vi "MasterAcquisitionFile_2P_Test.vi"() -> ()   [LabVIEW 2020]
uses:
  <vilib>/userDefined/High Color/IMAQdx.ctl
  <vilib>/vision/driver/IMAQdx.llb/IMAQdx Camera Control Mode.ctl
  <vilib>/vision/driver/IMAQdx.llb/IMAQdx Acquisition Mode.ctl
  <vilib>/vision/driver/IMAQdx.llb/IMAQdx Buffer Number Mode.ctl
  <vilib>/DAQmx/write.llb/DAQmx Write (Digital 1D Wfm NChan NSamp).vi
  <vilib>/DAQmx/read.llb/DAQmx Read (Analog 1D Wfm NChan NSamp).vi
  <vilib>/Waveform/DWDTOps.llb/DWDT Digital to Boolean Array.vi
  <vilib>/DAQmx/create/channels.llb/DAQmx Create Channel (DO-Digital Output).vi
  <vilib>/DAQmx/configure/timing.llb/DAQmx Timing (Sample Clock).vi
  <vilib>/Waveform/DWDTOps.llb/DWDT Boolean Array to Digital.vi
  <vilib>/Waveform/DWDTOps.llb/DWDT Uncompress Digital.vi
  <vilib>/DAQmx/miscellaneous.llb/DAQmx Fill In Error Info.vi
  <vilib>/DAQmx/create/channels.llb/DAQmx Create Channel (AI-Voltage-Basic).vi
  <vilib>/DAQmx/configure/trigger.llb/DAQmx Start Trigger (Digital Edge).vi
  <vilib>/DAQmx/create/channels.llb/DAQmx Create Channel (CO-Pulse Generation-Frequency).vi
  <vilib>/DAQmx/configure/timing.llb/DAQmx Timing (Implicit).vi
  <vilib>/DAQmx/read.llb/DAQmx Read (Digital 1D Bool 1Chan 1Samp).vi
  <vilib>/DAQmx/create/channels.llb/DAQmx Create Channel (DI-Digital Input).vi
  <vilib>/vision/driver/NI_Vision_Acquisition_Software.lvlib
  <resource>/objmgr/imaqdx.rc
  <resource>/objmgr/daqmx.rc
panel:
  in  "Analog Input Channels":tag="Dev2/ai0:3"
  out "Auditory":bool
  out "RPad":bool
  out "LPad":bool
  in  "Sol Stim Parameters":cluster{"Fs":dbl, "Samples":dbl}
  in  "LED Stim Parameters":cluster{"Fs":dbl, "Samples":dbl}
  in  "Generate Stimuli":bool=TRUE
  in  "Sol Duty Cycle (%)":dbl=50.0
  in  "Sol Freq":dbl=5.0
  in  "Sol Dur (s)":dbl=5.0
  in  "LED Duty Cycle (%)":dbl=10.0
  in  "LED Freq":dbl=10.0
  in  "LED Dur (s)":dbl=2.0
  out "Stimulus Order":digitalwaveform[](graph)=[{"t0"=timestamp(0 s since 1904-01-01), "dt"=5e-05, "Y"={"transitions"=[], "data"=array19221000x1[19221000 elements]}}, {"t0"=timestamp(0 s since 1904-01-01), "dt"=5e-05, "Y"={"transitions"=[], "data"=array19221000x1[19221000 elements]}}, {"t0"=timestamp(0 s since 1904-01-01), "dt"=5e-05, "Y"={"transitions"=[], "data"=array19221000x1[19221000 elements]}}]
  out "Solenoid Stim":digitalwaveform(graph)={"t0"=timestamp(0 s since 1904-01-01), "dt"=5e-05, "Y"={"transitions"=[], "data"=array100000x1[100000 elements]}}
  in  "Trial Offset (s)":dbl=45.0
  in  "Interstim (s)":dbl=45.0
  in  "Right Pad":dbl=1.0
  in  "Left Pad":dbl=1.0
  in  "Auditory":dbl=1.0
  in  "LED":dbl
  out "?":T1(plugin-control)
  out "MSCan Cam Fs":dbl(knob) scale=0.0..200.0
  out "MScan Cam":bool
  out "?":T1(plugin-control)
  in  "stop":bool
  out "?":T1(plugin-control)
  out "Behavior Cam Fs":dbl(knob) scale=0.0..200.0
  out "Behav Cam":bool
  out "Complete":bool
  out "Whisk Cam":bool
  out "Analog":bool
  out "MScan Trig":bool
  out "?":bool[](array[boolean])=[TRUE]
  out "Hexadecimal Data":u32=1 format="%x"
  out "Time Elapsed (Min)":cluster{dbl, dbl}(slide)={16.0, 0.0} scale=0.0..16.0 scale format="%#_2g"
  out "Whisker Camera":bool
  out "Analog Data":bool
  out "Analog Samples":i32=15417328
  in  "Device Analog Channel Labels":string[](array[string])=["forceSensor", "LPadSol", "RPadSol", "AudSol", "", "", "", ""]
  in  "?":cluster{"Analog Fs":u16}={"Analog Fs"=20000} {"Analog Fs" format="%0.0f"}
  in  "?":cluster{"WhiskerCam Fs":u16}={"WhiskerCam Fs"=150}
  out "Notes Size":i32=7
  out "Notes Reversed":string[](array[string])=["Experimenter", "Animal ID", "Isoflurane time", "Amplifier Gain", "Session ID", "Hemisphere", "Solenoid PSI"]
  out "Notes Array":string[](array[string])=["Solenoid PSI", "Hemisphere", "Session ID", "Amplifier Gain", "Isoflurane time", "Animal ID", "Experimenter"]
  in  "Notes:":T2={"Experimenter"="Kevin\n", "Animal ID"="T192", "Isoflurane time"="1145", "Amplifier Gain"="10000", "Session ID"="Imaging Session One", "Hemisphere"="RH", "Solenoid PSI"="10"}
  in  "Target Path":path=path "C:/Users/klt8/Documents" caption="Final Saved File Location"
  out "Dropped":u32(slide) caption="WhiskerCam" scale=0.0..150.0
  out "Current File Name":string="210517_13_39_46"
  in  "Time (min)":dbl(knob)=16.0 min=0.5 max=20.0 step=0.5 scale=0.0..20.0 scale format="%#_3g"
  in  "Temp Path":path=path "C:/Users/klt8/Documents/LabVIEW Temp Files" caption="Temporary File Path"
  out "Last Whisk Buffer":u32=115624
  out "Whisker Cam Fs":dbl(knob) scale=0.0..200.0 scale format="%#1_6g"
  # "Notes"
  # "Dropped Frames"
  # "LPAD"
  # "RPAD"
  # "AUD"
  # "Analog\nFs"
  # "Whisker\nFs"
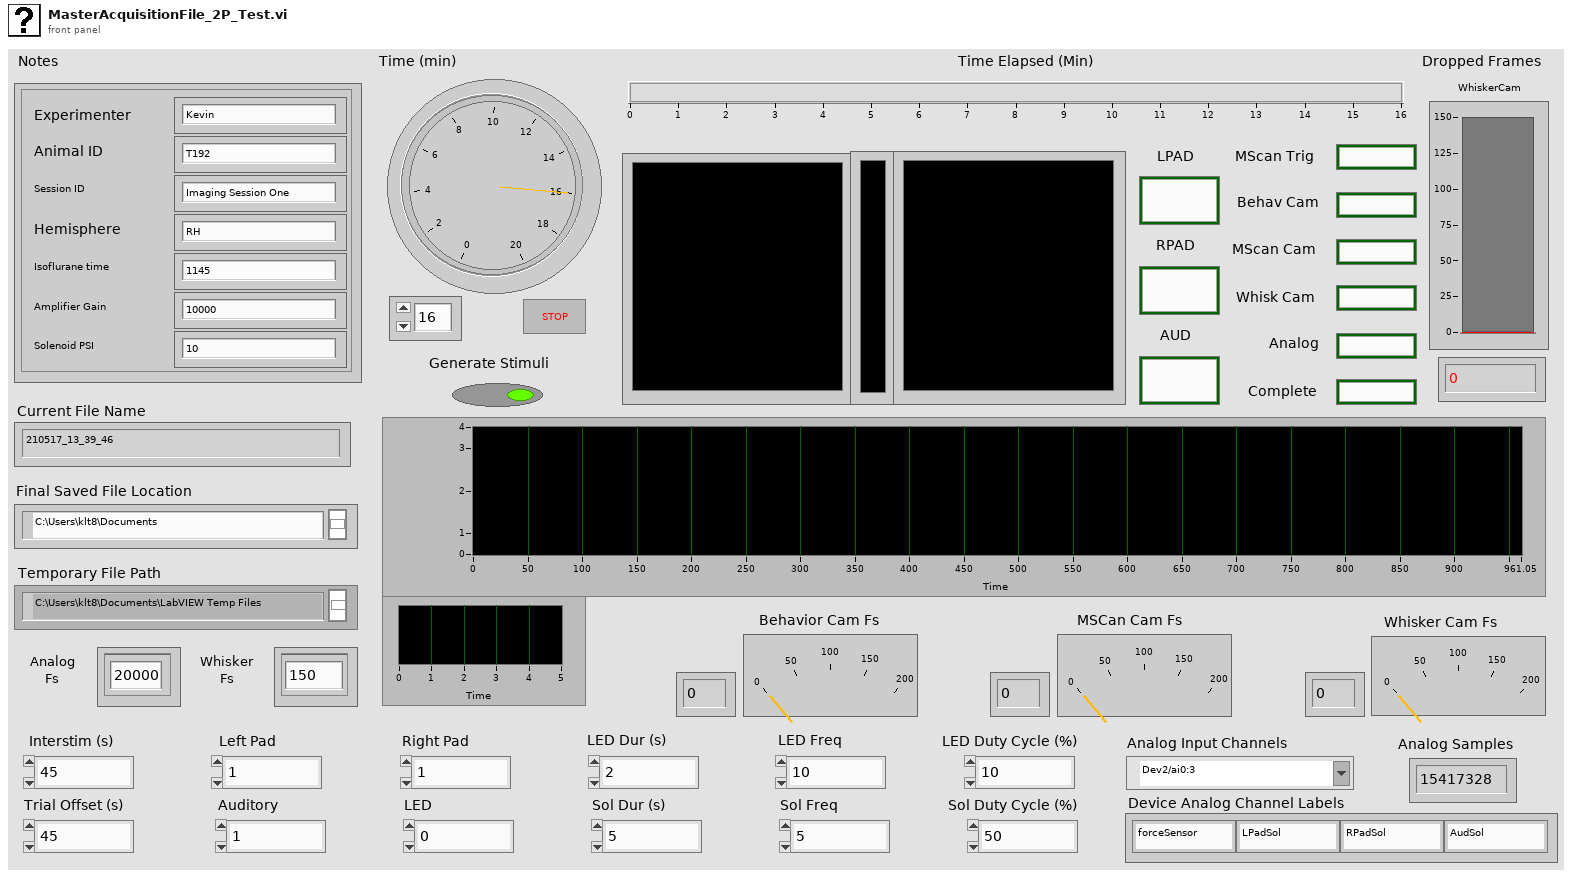
[diagram p1: front panel]
types:
  T1 = typedef "IMAQ Image.ctl" = refnum<image>
  T2 = cluster{"Experimenter":string, "Animal ID":string, "Isoflurane time":string, "Amplifier Gain":string, "Session ID":string, "Hemisphere":string, "Solenoid PSI":string}
  T3 = typedef "IMAQdx.ctl" = refnum<k21>
  T4 = typedef "NI_Vision_Acquisition_Software.lvlib/IMAQdx Camera Control Mode.ctl" = enum32{"Controller", "Listener"}
  T5 = enum16{"open", "open or create", "create or replace", "create", "open (read-only)"}
  T6 = enum16{"open", "replace", "create", "open or create", "replace or create", "replace or create with confirmation"}
  T7 = typedef "NI_Vision_Acquisition_Software.lvlib/IMAQdx Acquisition Mode.ctl" = enum32{"One Shot", "Continuous"}
  T8 = enum16{"big-endian, network order", "native, host order", "little-endian"}
  T9 = typedef "NI_Vision_Acquisition_Software.lvlib/IMAQdx Buffer Number Mode.ctl" = enum32{"Next", "Last", "Buffer Number", "Every", "Last New"}
  T10 = typedef "Image Type" = u32
  T11 = typedef "IMAQ AVI2 Refnum.ctl" = refnum<k20>
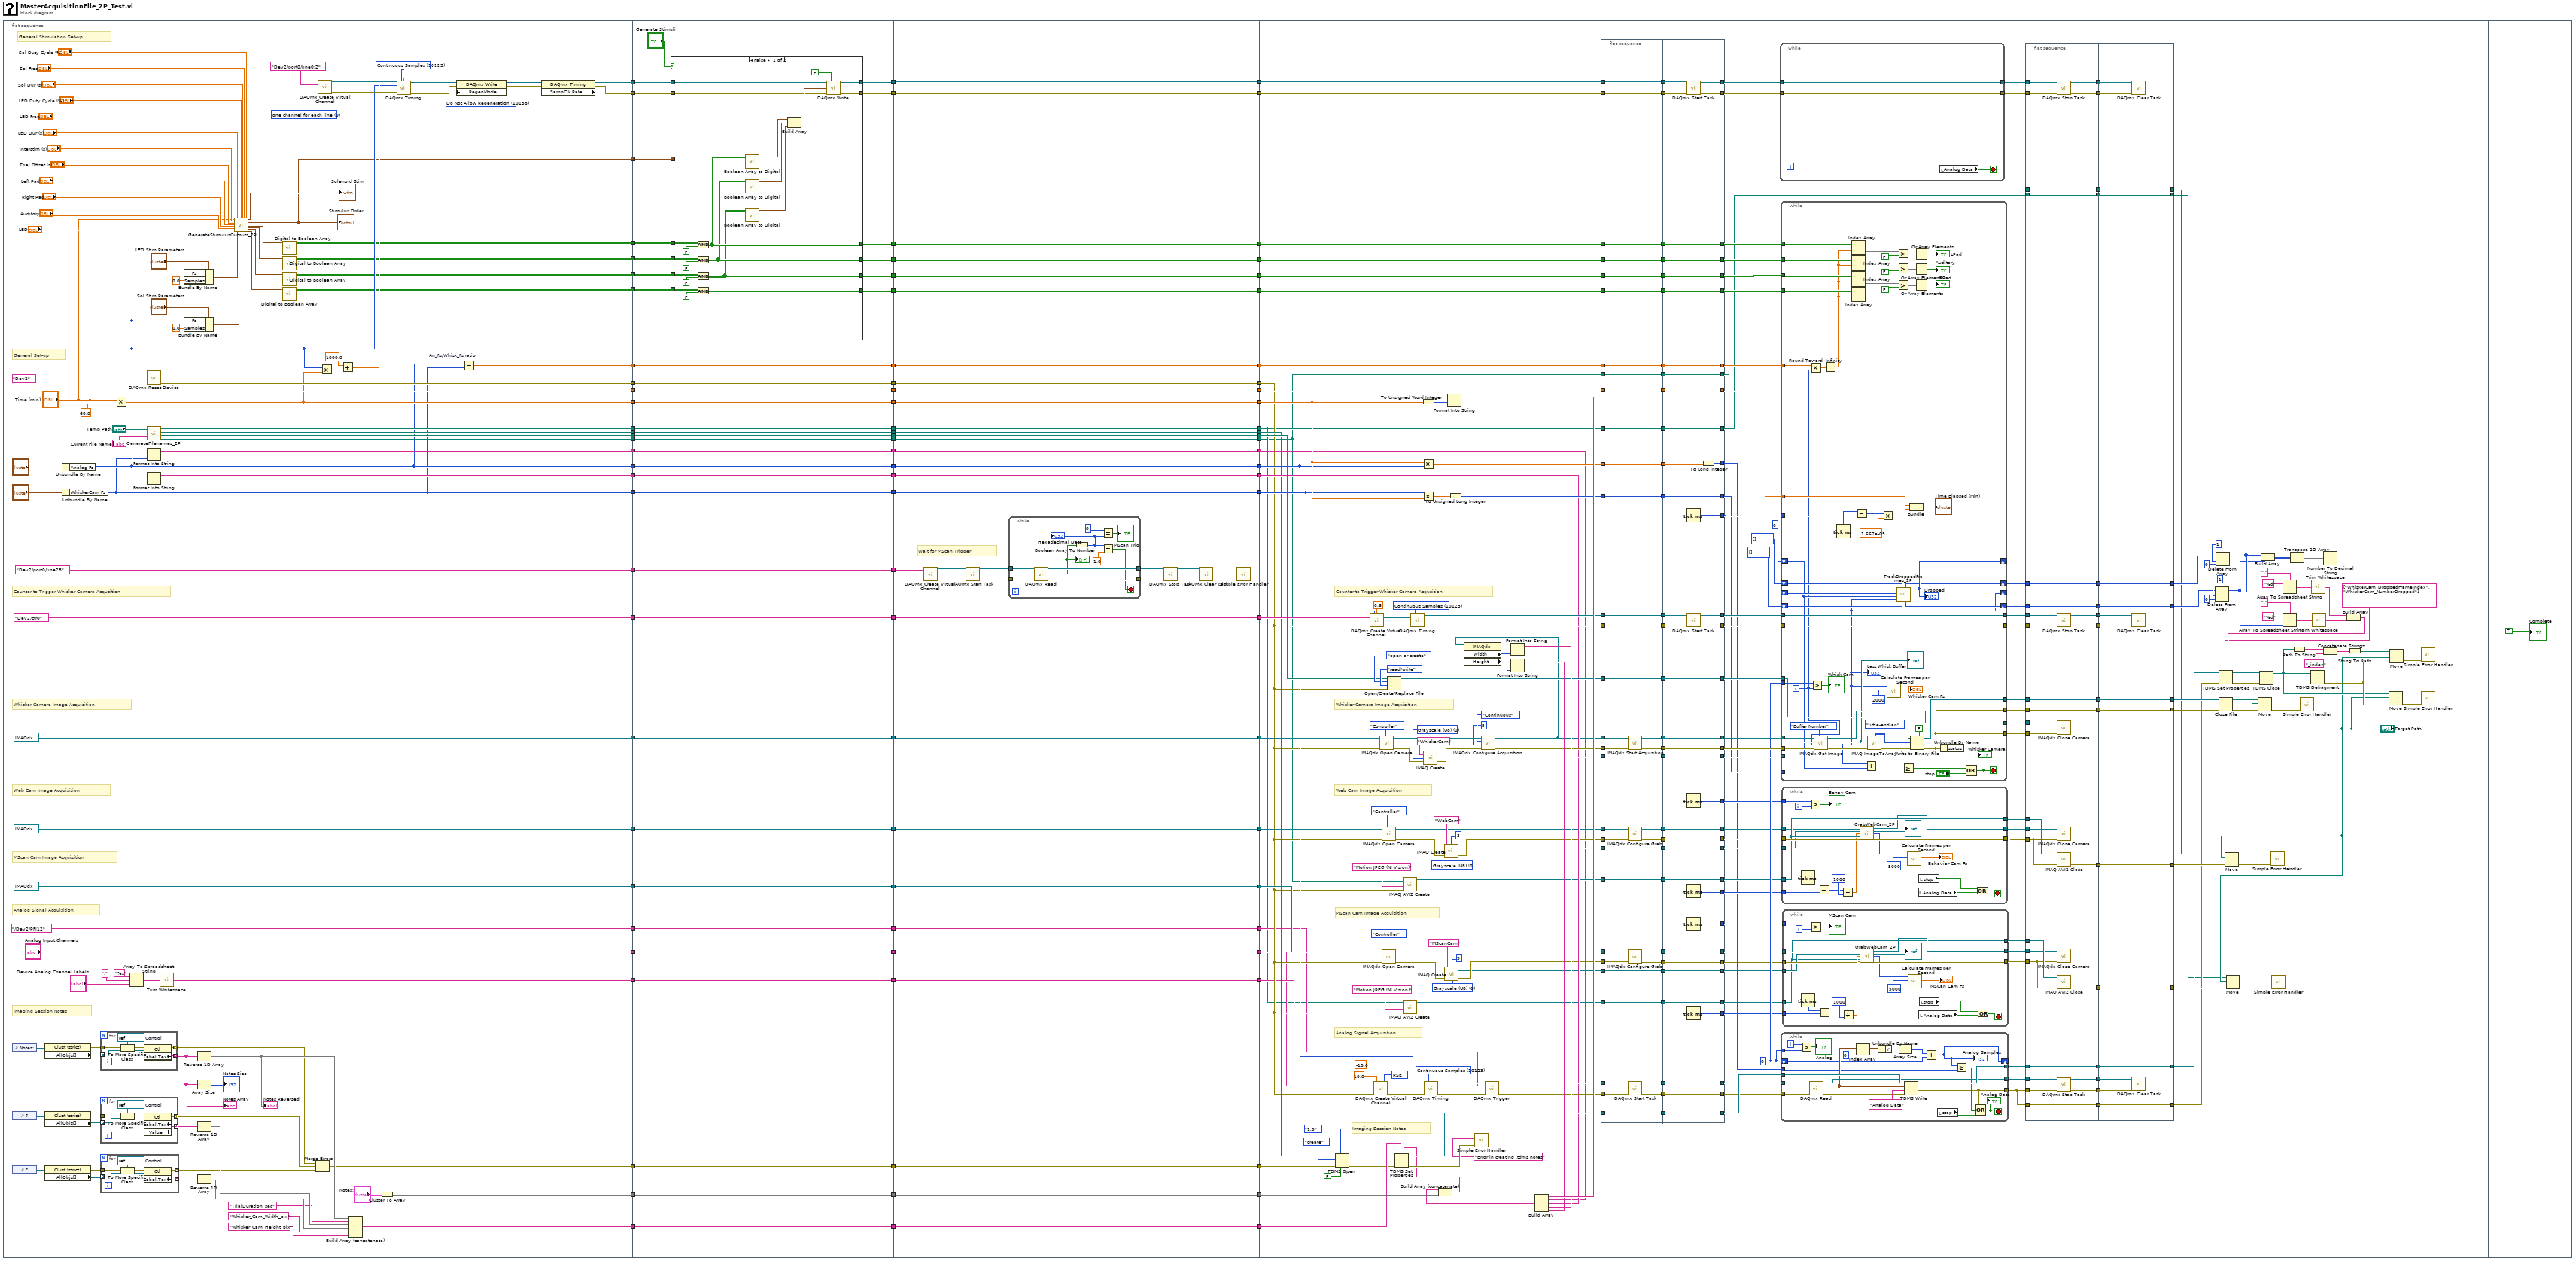
[diagram p0: block diagram]
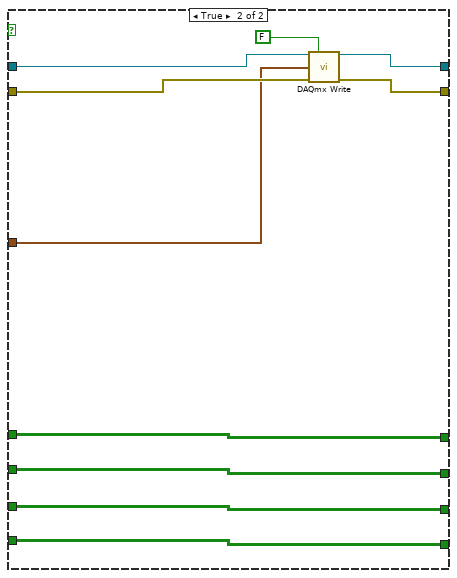
[diagram p2: hidden frame]
diagram:
  n1 = flat-sequence {
    tunnel: [tag "/Dev2/PFI12" ("Whisk Cam Trigger")] -> w62
    tunnel: [w109] -> w60
    tunnel: ["Time (min)"] -> w58
    tunnel: [w156] -> w56
    tunnel: [w155] -> w54
    tunnel: [w107] -> w52
    tunnel: [w106] -> w50
    tunnel: [w154] -> w48
    tunnel: [tag "Dev2/ctr0" ("Whisk Cam Counter")] -> w46
    tunnel: [w153] -> w44
    tunnel: ["Analog Input Channels"] -> w42
    tunnel: [T3 "cam1" ("Whisker Cam ID")] -> w40
    tunnel: [w152] -> w38
    tunnel: [w150] -> w36
    tunnel: [w151] -> w34
    tunnel: [T3 "cam2" ("WebCam ID")] -> w32
    tunnel: [tag "Dev2/port0/line28" ("MScan Trigger")] -> w30
    tunnel: [w147] -> w28
    tunnel: [w146] -> w26
    tunnel: [w145] -> w24
    tunnel: [T3 "cam7" ("WebCam ID 2")] -> w22
    tunnel: [w144] -> w20
    tunnel: [w105] -> w12
    tunnel: [w94] -> w10
    tunnel: [w93] -> w9
    tunnel: [w92] -> w8
    tunnel: [w91] -> w7
    tunnel: [w90] -> w6
    tunnel: [w89] -> w5
    tunnel: [w88] -> w4
    tunnel: w62 -> [w244]
    tunnel: [w244] -> w61
    tunnel: w60 -> [w243]
    tunnel: [w243] -> w59
    tunnel: w58 -> [w242]
    tunnel: [w242] -> w57
    tunnel: w56 -> [w241]
    tunnel: [w241] -> w55
    tunnel: w54 -> [w240]
    tunnel: [w240] -> w53
    tunnel: w52 -> [w239]
    tunnel: [w239] -> w51
    tunnel: w50 -> [w238]
    tunnel: [w238] -> w49
    tunnel: w48 -> [w237]
    tunnel: [w237] -> w47
    tunnel: w46 -> [w236]
    tunnel: [w236] -> w45
    tunnel: w44 -> [w235]
    tunnel: [w235] -> w43
    tunnel: w42 -> [w234]
    tunnel: [w234] -> w41
    tunnel: w40 -> [w233]
    tunnel: [w233] -> w39
    tunnel: w38 -> [w232]
    tunnel: [w232] -> w37
    tunnel: w36 -> [w231]
    tunnel: [w231] -> w35
    tunnel: w34 -> [w230]
    tunnel: [w230] -> w33
    tunnel: w32 -> [w229]
    tunnel: [w229] -> w31
    tunnel: w30 -> [w228]
    tunnel: [w228] -> w29
    tunnel: w28 -> [w227]
    tunnel: [w227] -> w27
    tunnel: w26 -> [w226]
    tunnel: [w226] -> w25
    tunnel: w24 -> [w225]
    tunnel: [w225] -> w23
    tunnel: w22 -> [w224]
    tunnel: [w224] -> w21
    tunnel: w20 -> [w223]
    tunnel: [w223] -> w19
    tunnel: [w214] -> w18
    tunnel: [w213] -> w17
    tunnel: [w212] -> w16
    tunnel: [w211] -> w15
    tunnel: [w210] -> w14
    tunnel: [w209] -> w13
    tunnel: w12 -> [w222]
    tunnel: [w222] -> w11
    tunnel: w10 -> [w221]
    tunnel: w9 -> [w220]
    tunnel: w8 -> [w219]
    tunnel: w7 -> [w218]
    tunnel: w6 -> [w217]
    tunnel: w5 -> [w216]
    tunnel: w4 -> [w215]
    tunnel: [w293] -> w87
    tunnel: [w304] -> w86
    tunnel: [w305] -> w85
    tunnel: [w306] -> w84
    tunnel: [w307] -> w83
    tunnel: [w294] -> w82
    tunnel: [w308] -> w81
    tunnel: [w309] -> w80
    tunnel: [w310] -> w79
    tunnel: [w311] -> w78
    tunnel: [w312] -> w77
    tunnel: [w313] -> w76
    tunnel: w61 -> [w278]
    tunnel: w59 -> [w313]
    tunnel: w57 -> [w312]
    tunnel: w55 -> [w311]
    tunnel: w53 -> [w310]
    tunnel: w51 -> [w309]
    tunnel: w49 -> [w308]
    tunnel: w47 -> [w294]
    tunnel: w45 -> [w307]
    tunnel: w43 -> [w276]
    tunnel: w41 -> [w277]
    tunnel: w39 -> [w306]
    tunnel: w37 -> [w305]
    tunnel: w35 -> [w304]
    tunnel: w33 -> [w293]
    tunnel: [w291] -> w75
    tunnel: w31 -> [w291]
    tunnel: w29 -> [w292]
    tunnel: w27 -> [w290]
    tunnel: [w290] -> w74
    tunnel: w25 -> [w289]
    tunnel: w23 -> [w288]
    tunnel: [w289] -> w73
    tunnel: [w288] -> w72
    tunnel: w21 -> [w287]
    tunnel: [w287] -> w71
    tunnel: w19 -> [w286]
    tunnel: [w286] -> w70
    tunnel: [w285] -> w69
    tunnel: w18 -> [w285]
    tunnel: [w284] -> w68
    tunnel: w17 -> [w284]
    tunnel: [w283] -> w67
    tunnel: w16 -> [w283]
    tunnel: [w282] -> w66
    tunnel: w15 -> [w282]
    tunnel: [w281] -> w65
    tunnel: w14 -> [w281]
    tunnel: w13 -> [w280]
    tunnel: [w280] -> w64
    tunnel: [w279] -> w63
    tunnel: w11 -> [w279]
    tunnel: [w278] -> w3
    tunnel: [w277] -> w2
    tunnel: [w276] -> w1
    tunnel: w87 -> [w468]
    tunnel: w86 -> [w474]
    tunnel: w85 -> [w416]
    tunnel: w84 -> [w473]
    tunnel: w83 -> [w472]
    tunnel: w82 -> [w471]
    tunnel: w81 -> [w441]
    tunnel: w80 -> [w431]
    tunnel: w79 -> [w470]
    tunnel: w78 -> [w430]
    tunnel: w77 -> [w465]
    tunnel: w76 -> [w469]
    tunnel: w75 -> [w456]
    tunnel: w74 -> [w348]
    tunnel: w73 -> [w437]
    tunnel: w72 -> [w435]
    tunnel: w71 -> [w418]
    tunnel: w70 -> [w350]
    tunnel: w69 -> [w370]
    tunnel: w68 -> [w368]
    tunnel: w67 -> [w374]
    tunnel: w66 -> [w373]
    tunnel: w65 -> [w372]
    tunnel: w64 -> [w371]
    tunnel: w63 -> [w389]
    tunnel: w3 -> [w354]
    tunnel: w2 -> [w352]
    tunnel: w1 -> [w353]
    frame #0 {
      w124 = 10158 items=["Allow Regeneration"=10097, "Do Not Allow Regeneration"=10158] ("RegenMode")
      w125 = 10123 items=["Finite Samples"=10178, "Continuous Samples"=10123, "Hardware Timed Single Point"=12522] ("sample mode")
      w128 = 0 items=["one channel for each line", "one channel for all lines"] ("line grouping")
      # "General Stimulation Set-up"
      # "MScan Cam Image Acquisition"
      # "General Set-up"
      # "Whisker Camera Image Acquisition"
      # "Imaging Session Notes"
      # "Counter to Trigger Whisker Camera Acqusition"
      # "Web Cam Image Acquisition"
      # "Analog Signal Acquisition"
      n2 = control-ref of="Notes:"() -> (w172:refnum<vi>)
      n3 = control-ref of="?"() -> (w170:refnum<vi>)
      n4 = control-ref of="?"() -> (w163:refnum<vi>)
      n5 = property class="Clust (strict)"(reference=w172) -> (error out=w171:errorcluster, "AllObjs[]"=w173:refnum<vi>[])  [unwired: 1 in, 1 out]
      n6 = property class="Clust (strict)"(reference=w170) -> (error out=w168:errorcluster, "AllObjs[]"=w169:refnum<vi>[])  [unwired: 1 in, 1 out]
      n7 = property class="Clust (strict)"(reference=w163) -> (error out=w164:errorcluster, "AllObjs[]"=w166:refnum<vi>[])  [unwired: 1 in, 1 out]
      n8 = Unbundle By Name("?") -> ("Analog Fs"=w107:u16)
      n9 = Unbundle By Name("?") -> ("WhiskerCam Fs"=w106:u16)
      n10 = for {
        tunnel: [w191] -> w178 mode=indexing
        tunnel: w173 -> [w190] mode=indexing
        tunnel: w171 -> [w189]
        tunnel: [w187] -> w177 mode=indexing
        w192 = refnum<vi> refnum  # Control
        n11 = To More Specific Class(target class=w192, reference=w190, error in=w189) -> (specific class reference=w193:refnum<vi>, error out=w188:errorcluster)
        n12 = property class="Ctl"(reference=w193, error in=w188) -> (error out=w187:errorcluster, "Label.Text"=w191:string)  [unwired: 1 out]
      }
      "Notes Array" <- w178
      n13 = for {
        tunnel: [w198] -> w167 mode=indexing
        tunnel: w169 -> [w197] mode=indexing
        tunnel: w168 -> [w196]
        tunnel: [w194] -> w176 mode=indexing
        w199 = refnum<vi> refnum  # Control
        n14 = To More Specific Class(target class=w199, reference=w197, error in=w196) -> (specific class reference=w200:refnum<vi>, error out=w195:errorcluster)
        n15 = property class="Ctl" props=["Label", "Text", "Value"](reference=w200, error in=w195) -> (error out=w194:errorcluster, "Label.Text"=w198:string)  [unwired: 2 out]
      }
      n16 = for {
        tunnel: [w205] -> w165 mode=indexing
        tunnel: w166 -> [w204] mode=indexing
        tunnel: w164 -> [w203]
        tunnel: [w201] -> w175 mode=indexing
        w206 = refnum<vi> refnum  # Control
        n17 = To More Specific Class(target class=w206, reference=w204, error in=w203) -> (specific class reference=w207:refnum<vi>, error out=w202:errorcluster)
        n18 = property class="Ctl"(reference=w207, error in=w202) -> (error out=w201:errorcluster, "Label.Text"=w205:string)  [unwired: 1 out]
      }
      n19 = Multiply(x="Time (min)", y=60.0) -> (x*y=w109:dbl)
      n20 = Array To Spreadsheet String(delimiter (Tab)=",", array="Device Analog Channel Labels", 3:"%s" ("format string")) -> (spreadsheet string=w180:string)
      n21 = call <vilib>:"DAQmx Reset Device.vi"("device in"=tag "Dev2" ("NI Board")) -> ("error out"=w152:errorcluster)  [unwired: 14 in]
      n22 = call "GenerateFilenames_2P.vi"("path"="Temp Path") -> ("WebCam Path"=w147:path, "Basler Path"=w150:path, "TDMS Path"=w145:path, "MScan Path"=w144:path, "Analog file name"=→"Current File Name":string)  [unwired: 2 in]
      n23 = Format Into String(w106) -> (resulting string=w156:string)  [unwired: 3 in, 1 out]
      n24 = Format Into String(w107) -> (resulting string=w155:string)  [unwired: 3 in, 1 out]
      n25 = call <vilib>:"Trim Whitespace.vi"("string"=w180) -> ("trimmed string"=w153:string)  [unwired: 1 in]
      n26 = Bundle By Name(cluster="LED Stim Parameters", "Fs"=w107, "Samples"=0.0) -> (w114:cluster{"Fs":dbl, "Samples":dbl})
      n27 = Bundle By Name(cluster="Sol Stim Parameters", "Fs"=w107, "Samples"=0.0) -> (w113:cluster{"Fs":dbl, "Samples":dbl})
      n28 = Reverse 1D Array(array=w178) -> (reversed array=w179:string[])
      "Notes Reversed" <- w179
      n29 = Array Size(array=w178) -> (size(s)=→"Notes Size":i32)
      n30 = Reverse 1D Array(array=w167) -> (reversed array=w185:string[])
      n31 = Reverse 1D Array(array=w165) -> (reversed array=w186:string[])
      n32 = call "GenerateStimulusOutputs_2P.vi"("Trial duration (min)"="Time (min)", "Rest duration(s)"="Interstim (s)", "trial offset (s)"="Trial Offset (s)", "Left Pad"="Left Pad", "Right Pad"="Right Pad", "Auditory"="Auditory", "LED"="LED", "LED Stim Duration (s)"="LED Dur (s)", "LED Stim Parameters"=w114, "LED Frequency"="LED Freq", "Sol Stim Parameters"=w113, "LED duty cycle (%)"="LED Duty Cycle (%)", "Sol Stim Duration (s)"="Sol Dur (s)", "Sol Frequency"="Sol Freq", "Sol Duty Cycle (%)"="Sol Duty Cycle (%)") -> ("Solenoid Stim Waveforms"=→"Solenoid Stim":digitalwaveform, "Stimulus Digital Outputs"=w90:digitalwaveform[], "Left Pad Out"=w103:digitalwaveform, "Auditory Out"=w130:digitalwaveform, "Right Pad Out"=w129:digitalwaveform, "LED Out"=w108:digitalwaveform)  [unwired: 7 in]
      "Stimulus Order" <- w90
      n33 = call-poly <vilib>:"Digital to Boolean Array.vi"("digital waveform"=w103) -> ("boolean array"=w89:bool[][])  [unwired: 9 in, 1 out]
      n34 = call-poly <vilib>:"Digital to Boolean Array.vi"("digital waveform"=w130) -> ("boolean array"=w92:bool[][])  [unwired: 9 in, 1 out]
      n35 = call-poly <vilib>:"Digital to Boolean Array.vi"("digital waveform"=w129) -> ("boolean array"=w91:bool[][])  [unwired: 9 in, 1 out]
      n36 = call-poly <vilib>:"Digital to Boolean Array.vi"("digital waveform"=w108) -> ("boolean array"=w88:bool[][])  [unwired: 9 in, 1 out]
      n37 = Merge Errors(w177, w176, w175) -> (w146:errorcluster)
      n38 = call-poly <vilib>:"DAQmx Create Virtual Channel.vi"("lines"=tag "Dev2/port0/line0:2", "line grouping"=w128) -> ("task out"=w127:refnum<k21>, "error out"=w126:errorcluster)  [unwired: 12 in]
      n39 = Multiply(x=w107, y=w109) -> (x*y=w112:dbl)
      n40 = Add(x=1000.0, y=w112) -> (x+y=w110:dbl)
      n41 = Build Array (concatenate)(w179, "TrialDuration_sec", w185, w186, "Whisker_Cam_Width_pix", "Whisker_Cam_Height_pix") -> (w151:string[])
      n42 = Cluster To Array(cluster="Notes:") -> (array=w154:string[])
      n43 = call-poly <vilib>:"DAQmx Timing.vi"("task/channels in"=w127, "sample mode"=w125, "samples per channel"=w110, "rate"=w107, "error in"=w126) -> ("task out"=w121:refnum<k21>, "error out"=w120:errorcluster)  [unwired: 9 in]
      n44 = property class="DAQmx Write"(reference=w121, error in=w120, "RegenMode"=w124) -> (reference out=w122:refnum<k21>, error out=w123:errorcluster)
      n45 = Divide "An_Fs/Whisk_Fs ratio"(x=w107, y=w106) -> (x/y=w105:dbl)
      n46 = property class="DAQmx Timing" props=["SampClk.Rate"](reference=w122, error in=w123) -> (reference out=w94:refnum<k21>, error out=w93:errorcluster)  [unwired: 1 out]
    }
    frame #1 {
      n47 = case shown="False" "Generate Stimuli" {
        tunnel: w221 -> [w252 w275]
        tunnel: w220 -> [w251 w274]
        tunnel: [w249 w273] -> w214
        tunnel: [w250 w272] -> w213
        tunnel: w219 -> [w264 w271]
        tunnel: w218 -> [w265 w270]
        tunnel: [w248 w268] -> w212
        tunnel: [w247 w271] -> w211
        tunnel: [w246 w270] -> w210
        tunnel: [w258 w267] -> w209
        tunnel: w217 -> [_ w269]
        tunnel: w216 -> [w259 w268]
        tunnel: w215 -> [w257 w267]
        frame False {
          n48 = Compound Arithmetic op=AND(w259, FALSE) -> (w248:bool[][])
          n49 = Compound Arithmetic op=AND(w264, FALSE) -> (w247:bool[][])
          n50 = Compound Arithmetic op=AND(w265, FALSE) -> (w246:bool[][])
          n51 = Compound Arithmetic op=AND(w257, FALSE) -> (w258:bool[][])
          n52 = call-poly <vilib>:"Boolean Array to Digital.vi"("boolean array"=w248) -> ("digital waveform"=w255:digitalwaveform)  [unwired: 9 in, 1 out]
          n53 = call-poly <vilib>:"Boolean Array to Digital.vi"("boolean array"=w247) -> ("digital waveform"=w254:digitalwaveform)  [unwired: 9 in, 1 out]
          n54 = call-poly <vilib>:"Boolean Array to Digital.vi"("boolean array"=w246) -> ("digital waveform"=w245:digitalwaveform)  [unwired: 9 in, 1 out]
          n55 = Build Array(w255, w254, w245) -> (w253:digitalwaveform[])
          n56 = call-poly <vilib>:"DAQmx Write.vi"("task/channels in"=w252, "auto start"=FALSE, "data"=w253, "error in"=w251) -> ("task out"=w249:refnum<k21>, "error out"=w250:errorcluster)  [unwired: 9 in, 1 out]
        }
        frame True {
          n57 = call-poly <vilib>:"DAQmx Write.vi"("task/channels in"=w275, "auto start"=FALSE, "data"=w269, "error in"=w274) -> ("task out"=w273:refnum<k21>, "error out"=w272:errorcluster)  [unwired: 9 in, 1 out]
        }
      }
    }
    frame #2 {
      # "Wait for MScan Trigger"
      n58 = call-poly <vilib>:"DAQmx Create Virtual Channel.vi"("lines"=w292) -> ("task out"=w299:refnum<k21>, "error out"=w300:errorcluster)  [unwired: 13 in]
      n59 = call <vilib>:"DAQmx Start Task.vi"("task/channels in"=w299, "error in"=w300) -> ("task out"=w303:refnum<k21>, "error out"=w302:errorcluster)  [unwired: 12 in]
      n60 = while {
        tunnel: w303 -> [w323]
        tunnel: w302 -> [w322]
        tunnel: [w320] -> w297
        tunnel: [w321] -> w298
        stop <- w315 stop-if-true
        n61 = call-poly <vilib>:"DAQmx Read.vi"("task/channels in"=w323, "error in"=w322) -> ("task out"=w321:refnum<k21>, "data"=w319:bool[], "error out"=w320:errorcluster)  [unwired: 11 in]
        "?" <- w319
        n62 = Boolean Array To Number(Boolean array=w319) -> (number=w314:u32)
        "Hexadecimal Data" <- w314
        n63 = Equal?(x=w314, y=u32 0) -> (x = y?=→"MScan Trig":bool)
        n64 = Equal?(x=w314, y=1.0) -> (x = y?=w315:bool)
      }
      n65 = call <vilib>:"DAQmx Stop Task.vi"("task/channels in"=w298, "error in"=w297) -> ("task out"=w296:refnum<k21>, "error out"=w295:errorcluster)  [unwired: 12 in]
      n66 = call <vilib>:"DAQmx Clear Task.vi"("task in"=w296, "error in"=w295) -> ("error out"=w301:errorcluster)  [unwired: 13 in]
      n67 = call <vilib>:"Simple Error Handler.vi"("error in (no error)"=w301) -> ()  [unwired: 4 in, 5 out]
    }
    frame #3 {
      w421 = T10 0 items=["Grayscale (U8)", "Grayscale (I16)", "Grayscale (SGL)", "Complex (CSG)", "RGB (U32)", "HSL (U32)", "RGB (U64)", "Grayscale (U16)"] ("Image Type")
      w460 = T10 0 items=["Grayscale (U8)", "Grayscale (I16)", "Grayscale (SGL)", "Complex (CSG)", "RGB (U32)", "HSL (U32)", "RGB (U64)", "Grayscale (U16)"] ("Image Type")
      w448 = u32 0 ("y")
      w483 = 10123 items=["Finite Samples"=10178, "Continuous Samples"=10123, "Hardware Timed Single Point"=12522] ("sample mode")
      w482 = 10083 items=["default"=-1, "RSE"=10083, "NRSE"=10078, "Differential"=10106, "Pseudodifferential"=12529] ("input terminal configuration")
      w484 = 10123 items=["Finite Samples"=10178, "Continuous Samples"=10123, "Hardware Timed Single Point"=12522] ("sample mode")
      w480 = T10 0 items=["Grayscale (U8)", "Grayscale (I16)", "Grayscale (SGL)", "Complex (CSG)", "RGB (U32)", "HSL (U32)", "RGB (U64)", "Grayscale (U16)"] ("Image Type")
      # "MScan Cam Image Acquisition"
      # "Whisker Camera Image Acquisition"
      # "Imaging Session Notes"
      # "Counter to Trigger Whisker Camera Acqusition"
      # "Web Cam Image Acquisition"
      # "Analog Signal Acquisition"
      n68 = TDMS Open(6:FALSE ("disable buffering? (T)"), 7:enum16{"1.0", "2.0"}."1.0" ("file format version (2.0)"), 8:w437, 10:T5."create" ("operation (0:open)"), 11:w435) -> (0:w434:errorcluster, 3:w433:refnum<k34>)  [unwired: 2 in]
      n69 = call-poly <vilib>:"DAQmx Create Virtual Channel.vi"("frequency"=w441, "duty cycle"=0.6, "counter"=w472, "error in"=w416) -> ("task out"=w507:refnum<k21>, "error out"=w508:errorcluster)  [unwired: 10 in]
      n70 = call-poly <vilib>:"DAQmx Create Virtual Channel.vi"("maximum value"=10.0, "minimum value"=-10.0, "input terminal configuration"=w482, "physical channels"=w352, "name to assign"=w353, "error in"=w416) -> ("task out"=w515:refnum<k21>, "error out"=w516:errorcluster)  [unwired: 8 in]
      n71 = call <vilib>:"IMAQdx Open Camera.vi"("Camera Control Mode"=IMAQdx_Camera_Control_Mode."Controller", "error in"=w416, "Session In"=w473) -> ("error out"=w505:errorcluster, "Session Out"=w504:T3)  [unwired: 7 in]
      n72 = call <vilib>:"IMAQdx Open Camera.vi"("Camera Control Mode"=IMAQdx_Camera_Control_Mode."Controller", "error in"=w416, "Session In"=w456) -> ("error out"=w457:errorcluster, "Session Out"=w455:T3)  [unwired: 7 in]
      n73 = call <vilib>:"IMAQdx Open Camera.vi"("Camera Control Mode"=IMAQdx_Camera_Control_Mode."Controller", "error in"=w416, "Session In"=w418) -> ("error out"=w419:errorcluster, "Session Out"=w413:T3)  [unwired: 7 in]
      n74 = Open/Create/Replace File(file path (use dialog)=w474, error in=w416, operation (0:open)=T6."open or create", access (0:read/write)=enum16{"read/write", "read-only", "write-only"}."read/write") -> (refnum out=w514:refnum<file>)  [unwired: 2 in, 2 out]
      n75 = call "IMAQ AVI2 Create"("error in (no error)"=w416, "Codec"="Motion JPEG (NI Vision)", "AVI Path"=w348) -> ("AVI Refnum"=w443:T11)  [unwired: 7 in, 1 out]
      n76 = call "IMAQ AVI2 Create"("error in (no error)"=w416, "Codec"="Motion JPEG (NI Vision)", "AVI Path"=w350) -> ("AVI Refnum"=w409:T11)  [unwired: 7 in, 1 out]
      n77 = call-poly <vilib>:"DAQmx Timing.vi"("task/channels in"=w507, "sample mode"=w484, "error in"=w508) -> ("task out"=w524:refnum<k21>, "error out"=w525:errorcluster)  [unwired: 11 in]
      n78 = Multiply(x=w469, y=w431) -> (x*y=w547:dbl)
      n79 = Multiply(x=w441, y=w469) -> (x*y=w548:dbl)
      n80 = To Unsigned Word Integer(number=w469) -> (unsigned 16bit integer=w537:u16)
      n81 = call "IMAQ Create"("Image Name"="WhiskerCam", "Image Type"=w480, "error in (no error)"=w505) -> ("New Image"=w540:T1, "error out"=w506:errorcluster)  [unwired: 2 in]
      n82 = call-poly <vilib>:"DAQmx Timing.vi"("task/channels in"=w515, "sample mode"=w483, "rate"=w431, "error in"=w516) -> ("task out"=w517:refnum<k21>, "error out"=w518:errorcluster)  [unwired: 10 in]
      n83 = call "IMAQ Create"("Border Size"=3, "Image Name"="WebCam", "Image Type"=w460, "error in (no error)"=w457) -> ("New Image"=w453:T1, "error out"=w454:errorcluster)  [unwired: 1 in]
      n84 = call "IMAQ Create"("Border Size"=3, "Image Name"="MScanCam", "Image Type"=w421, "error in (no error)"=w419) -> ("New Image"=w403:T1, "error out"=w414:errorcluster)  [unwired: 1 in]
      n85 = Format Into String(w537) -> (resulting string=w556:string)  [unwired: 3 in, 1 out]
      n86 = To Unsigned Long Integer(number=w548) -> (unsigned 32bit integer=w549:u32)
      n87 = call <vilib>:"IMAQdx Configure Acquisition.vi"("error in"=w506, "Number of Buffers"=u32 5, "Continuous?"=IMAQdx_Acquisition_Mode."Continuous", "Session In"=w504) -> ("error out"=w509:errorcluster, "Session Out"=w432:T3)  [unwired: 6 in]
      n88 = property class="IMAQdx"(reference=w432) -> ("Width"=w538:u32, "Height"=w539:u32)  [unwired: 1 in, 2 out]
      n89 = call-poly <vilib>:"DAQmx Trigger.vi"("task/channels in"=w517, "source"=w354, "error in"=w518) -> ("task out"=w519:refnum<k21>, "error out"=w520:errorcluster)  [unwired: 11 in]
      n90 = Format Into String(w538) -> (resulting string=w555:string)  [unwired: 3 in, 1 out]
      n91 = Format Into String(w539) -> (resulting string=w554:string)  [unwired: 3 in, 1 out]
      n92 = Build Array(w556, w430, w470, w555, w554) -> (w428:string[])
      n93 = Build Array (concatenate)(w471, w428) -> (w475:string[])
      n94 = TDMS Set Properties(5:w475, 7:w468, 8:w434, 11:w433) -> (0:w536:errorcluster, 3:w535:refnum<k34>)  [unwired: 2 in, 2 out]
      n95 = call <vilib>:"Simple Error Handler.vi"("error source (\" \")"="Error in creating .tdms notes" ("error source (\" \")"), "error in (no error)"=w536) -> ()  [unwired: 3 in, 5 out]
      n96 = flat-sequence {
        tunnel: w432 -> [w717]
        tunnel: w509 -> [w716]
        tunnel: [w715] -> w567
        tunnel: [w714] -> w566
        tunnel: [w713] -> w565
        tunnel: w540 -> [w713]
        tunnel: [w712] -> w564
        tunnel: w514 -> [w712]
        tunnel: w519 -> [w711]
        tunnel: w520 -> [w710]
        tunnel: [w709] -> w563
        tunnel: [w708] -> w562
        tunnel: [w707] -> w561
        tunnel: w535 -> [w707]
        tunnel: w524 -> [w706]
        tunnel: [w706] -> w560
        tunnel: w525 -> [w705]
        tunnel: [w705] -> w559
        tunnel: w547 -> [w704]
        tunnel: [w704] -> w558
        tunnel: w549 -> [w703]
        tunnel: [w703] -> w557
        tunnel: w465 -> [w702]
        tunnel: [w702] -> w464
        tunnel: w455 -> [w701]
        tunnel: w454 -> [w700]
        tunnel: w453 -> [w699]
        tunnel: [w699] -> w452
        tunnel: [w698] -> w451
        tunnel: [w697] -> w450
        tunnel: [w696] -> w444
        tunnel: w443 -> [w696]
        tunnel: w414 -> [w692]
        tunnel: w413 -> [w695]
        tunnel: [w694] -> w412
        tunnel: [w693] -> w411
        tunnel: [w691] -> w410
        tunnel: w409 -> [w691]
        tunnel: [w690] -> w404
        tunnel: w403 -> [w690]
        tunnel: [w689] -> w398
        tunnel: w374 -> [w689]
        tunnel: [w688] -> w397
        tunnel: w373 -> [w688]
        tunnel: [w687] -> w396
        tunnel: w372 -> [w687]
        tunnel: [w686] -> w395
        tunnel: w371 -> [w686]
        tunnel: [w685] -> w390
        tunnel: w389 -> [w685]
        tunnel: w370 -> [w683]
        tunnel: [w684] -> w369
        tunnel: w368 -> [w684]
        tunnel: [w683] -> w367
        tunnel: [w682] -> w351
        tunnel: w350 -> [w682]
        tunnel: [w681] -> w349
        tunnel: w348 -> [w681]
        tunnel: [w749] -> w466
        tunnel: [w748] -> w467
        tunnel: [w756] -> w510
        tunnel: w567 -> [w756]
        tunnel: [w755] -> w511
        tunnel: w566 -> [w755]
        tunnel: [w754] -> w512
        tunnel: w565 -> [w754]
        tunnel: [w753] -> w513
        tunnel: w564 -> [w753]
        tunnel: [w752] -> w522
        tunnel: w563 -> [w752]
        tunnel: [w751] -> w521
        tunnel: w562 -> [w751]
        tunnel: [w750] -> w523
        tunnel: w561 -> [w750]
        tunnel: w560 -> [w745]
        tunnel: w559 -> [w747]
        tunnel: w558 -> [w736]
        tunnel: w557 -> [w746]
        tunnel: [w746] -> w427
        tunnel: [w744] -> w503
        tunnel: w464 -> [w743]
        tunnel: [w743] -> w463
        tunnel: [w742] -> w447
        tunnel: w452 -> [w742]
        tunnel: [w741] -> w445
        tunnel: w451 -> [w741]
        tunnel: [w740] -> w446
        tunnel: w450 -> [w740]
        tunnel: [w739] -> w440
        tunnel: w444 -> [w738]
        tunnel: [w738] -> w442
        tunnel: [w737] -> w439
        tunnel: [w735] -> w426
        tunnel: [w734] -> w406
        tunnel: w412 -> [w734]
        tunnel: [w733] -> w405
        tunnel: w411 -> [w733]
        tunnel: [w732] -> w400
        tunnel: w410 -> [w732]
        tunnel: [w731] -> w408
        tunnel: [w730] -> w407
        tunnel: w404 -> [w729]
        tunnel: [w729] -> w402
        tunnel: w398 -> [w728]
        tunnel: [w728] -> w394
        tunnel: [w727] -> w393
        tunnel: w397 -> [w727]
        tunnel: w396 -> [w726]
        tunnel: [w726] -> w392
        tunnel: w395 -> [w725]
        tunnel: [w725] -> w391
        tunnel: [w724] -> w388
        tunnel: w390 -> [w724]
        tunnel: [w723] -> w387
        tunnel: [w722] -> w386
        tunnel: w369 -> [w721]
        tunnel: w367 -> [w720]
        tunnel: w351 -> [w719]
        tunnel: [w719] -> w326
        tunnel: w349 -> [w718]
        tunnel: [w718] -> w327
        frame #0 {
          n97 = call <vilib>:"IMAQdx Start Acquisition.vi"("error in"=w716, "Session In"=w717) -> ("error out"=w714:errorcluster, "Session Out"=w715:T3)  [unwired: 8 in]
          n98 = call <vilib>:"IMAQdx Configure Grab.vi"("error in"=w700, "Session In"=w701) -> ("error out"=w697:errorcluster, "Session Out"=w698:T3)  [unwired: 8 in]
          n99 = call <vilib>:"IMAQdx Configure Grab.vi"("error in"=w692, "Session In"=w695) -> ("error out"=w693:errorcluster, "Session Out"=w694:T3)  [unwired: 8 in]
          n100 = call <vilib>:"DAQmx Start Task.vi"("task/channels in"=w711, "error in"=w710) -> ("task out"=w709:refnum<k21>, "error out"=w708:errorcluster)  [unwired: 12 in]
        }
        frame #1 {
          n101 = call <vilib>:"DAQmx Start Task.vi"("task/channels in"=w720, "error in"=w721) -> ("task out"=w723:refnum<k21>, "error out"=w722:errorcluster)  [unwired: 12 in]
          n102 = Tick Count (ms)() -> (millisecond timer value=w744:u32)
          n103 = call <vilib>:"DAQmx Start Task.vi"("task/channels in"=w745, "error in"=w747) -> ("task out"=w749:refnum<k21>, "error out"=w748:errorcluster)  [unwired: 12 in]
          n104 = Tick Count (ms)() -> (millisecond timer value=w739:u32)
          n105 = Tick Count (ms)() -> (millisecond timer value=w737:u32)
          n106 = Tick Count (ms)() -> (millisecond timer value=w730:u32)
          n107 = Tick Count (ms)() -> (millisecond timer value=w731:u32)
          n108 = To Long Integer(number=w736) -> (32bit integer=w735:i32)
        }
      }
      n109 = while {
        tunnel: w387 -> [w616]
        tunnel: [w614] -> w382
        tunnel: w386 -> [w614]
        tunnel: [w616] -> w383
        stop <- w615 stop-if-true
        n110 = local read "Analog Data"() -> (w615:bool)
      }
      n111 = while {
        tunnel: [w802] -> w365
        tunnel: [w786] -> w340
        tunnel: [w810] -> w337
        tunnel: w510 -> [w809]
        tunnel: w511 -> [w808]
        tunnel: w512 -> [w807]
        tunnel: w513 -> [w780]
        shift-right: [w760] -> _
        shift-left: _ -> [w806]
        shift-right: [w805] -> _
        shift-left: u32 0 ("New Lost") -> [w801]
        shift-right: [w804] -> w346
        shift-left: u32[] [] ("NewBuffNum") -> [w759]
        shift-right: [w803] -> w343
        shift-left: u32[] [] ("NewNumLost") -> [w795]
        tunnel: w427 -> [w799]
        tunnel: w503 -> [w790]
        tunnel: w463 -> [w788]
        tunnel: [w786] -> w366
        tunnel: w448 -> [w785]
        tunnel: w467 -> [w783]
        tunnel: w466 -> [w782]
        tunnel: [w783] -> w380
        tunnel: [w782] -> w381
        tunnel: w394 -> [w766]
        tunnel: w393 -> [w765]
        tunnel: w392 -> [w764]
        tunnel: w391 -> [w763]
        tunnel: w388 -> [w761]
        i -> [w757]
        stop <- w796 stop-if-true
        n112 = Multiply(x=w761, y=w757) -> (x*y=w762:dbl)
        n113 = Greater?(x=w757, y=w785) -> (0:→"Whisk Cam":bool)
        n114 = call <vilib>:"IMAQdx Get Image.vi"("Buffer Number Mode (Next)"=IMAQdx_Buffer_Number_Mode."Buffer Number", "error in"=w808, "Buffer Number In"=w757, "Image In"=w807, "Session In"=w809) -> ("error out"=w816:errorcluster, "Buffer Number Out"=w760:u32, "Image Out"=w779:T1, "Session Out"=w802:T3)  [unwired: 3 in]
        "Last Whisk Buffer" <- w760
        "?" <- w779
        n115 = Round Toward -Infinity(1:w762) -> (0:w758:dbl)
        n116 = Tick Count (ms)() -> (millisecond timer value=w791:u32)
        n117 = Index Array(array=w766, index (row)=w758) -> (element=w772:bool[])  [unwired: 1 in]
        n118 = Index Array(array=w765, index (row)=w758) -> (element=w770:bool[])  [unwired: 1 in]
        n119 = Index Array(array=w764, index (row)=w758) -> (element=w768:bool[])  [unwired: 1 in]
        n120 = Index Array(array=w763, index (row)=w758) -> ()  [unwired: 1 in, 1 out]
        n121 = Subtract(x=w791, y=w790) -> (x-y=w794:u32)
        n122 = Add(x=w760, y=w801) -> (x+y=w800:u32)
        n123 = call "IMAQ ImageToArray"("error in (no error)"=w816, "Image"=w779) -> ("error out"=w815:errorcluster, "Image Pixels (U8)"=w814:u8[][])  [unwired: 2 in, 3 out]
        n124 = Multiply(x=w794, y=1.667e-05) -> (x*y=w793:dbl)
        n125 = call <vilib>:"Calculate Frames per Second.vi"("Update Interval (ms)"=u32 2000, "Buffer Number"=w760) -> ("Processed Frames/s"=→"Whisker Cam Fs":dbl)  [unwired: 7 in, 2 out]
        n126 = Greater?(x=w772, y=FALSE ("Boolean")) -> (0:w771:bool[])
        n127 = Greater?(x=w770, y=FALSE ("Boolean")) -> (0:w769:bool[])
        n128 = Greater?(x=w768, y=FALSE ("Boolean")) -> (0:w767:bool[])
        n129 = call "TrackDroppedFrames_2P.vi"("NumLost"=w795, "BuffNum"=w759, "Curr Buffer"=w760, "Prev Lost"=w801, "Prev Buffer"=w806) -> ("New Lost"=w805:u32, "NewNumLost"=w803:u32[], "NewBuffNum"=w804:u32[])  [unwired: 4 in]
        "Dropped" <- w805
        n130 = Greater Or Equal?(x=w800, y=w799) -> (x >= y?=w797:bool)
        n131 = Bundle("Time (min)"=w788, w793) -> (→"Time Elapsed (Min)":cluster{"Time (min)":dbl, dbl})  [unwired: 1 in]
        n132 = Write to Binary File(file (use dialog)=w780, data=w814, error in=w815, 5:FALSE ("prepend array or string size? (T)"), 9:T8."little-endian" ("byte order (0:big-endian, network order)")) -> (refnum out=w810:refnum<file>, error out=w786:errorcluster)  [unwired: 1 in, 1 out]
        n133 = Or Array Elements(Boolean array=w771) -> (logical OR=→"LPad":bool)
        n134 = Or Array Elements(Boolean array=w769) -> (logical OR=→"Auditory":bool)
        n135 = Or Array Elements(Boolean array=w767) -> (logical OR=→"RPad":bool)
        n136 = Unbundle By Name(w786) -> ("status"=w798:bool)
        n137 = Compound Arithmetic op=OR(w798, w797, "stop") -> (w796:bool)
        "Whisker Camera" <- w796
      }
      n138 = while {
        tunnel: w521 -> [w680]
        tunnel: w522 -> [w679]
        tunnel: w523 -> [w678]
        tunnel: [w677] -> w334
        tunnel: [w665] -> w331
        tunnel: [w676] -> w375
        shift-right: [w669] -> _
        shift-left: w448 -> [w670]
        tunnel: w448 -> [w661]
        tunnel: w426 -> [w659]
        i -> [w662]
        stop <- w666 stop-if-true
        n139 = Greater?(x=w662, y=w661) -> (0:→"Analog":bool)
        n140 = call-poly <vilib>:"DAQmx Read.vi"("task/channels in"=w679, "error in"=w680) -> ("task out"=w676:refnum<k21>, "data"=w674:waveform(dbl)[], "error out"=w668:errorcluster)  [unwired: 11 in]
        n141 = Index Array(array=w674, index=0) -> (element=w672:waveform(dbl))
        n142 = Unbundle By Name(w672) -> ("Y"=w671:dbl[])
        n143 = Array Size(array=w671) -> (size(s)=w664:i32)
        n144 = TDMS Write(0:w678, 5:"Analog Data" ("group name in (Untitled)"), 9:w674, 11:w668) -> (4:w677:refnum<k34>, 15:w665:errorcluster)  [unwired: 2 in, 2 out]
        n145 = Add(x=w664, y=w670) -> (x+y=w669:u32)
        "Analog Samples" <- w669
        n146 = local read "stop"() -> (w660:bool)
        n147 = Greater Or Equal?(x=w669, y=w659) -> (x >= y?=w667:bool)
        n148 = Compound Arithmetic op=OR(w660, w665, w667) -> (w666:bool)
        "Analog Data" <- w666
      }
      n149 = while {
        tunnel: w447 -> [w645]
        tunnel: w445 -> [w644]
        tunnel: w446 -> [w648]
        tunnel: w442 -> [w647]
        tunnel: [w638] -> w362
        tunnel: [w649] -> w364
        tunnel: [w647] -> w363
        tunnel: w440 -> [w651]
        tunnel: w439 -> [w650]
        i -> [w652]
        stop <- w640 stop-if-true
        n150 = Tick Count (ms)() -> (millisecond timer value=w656:u32)
        n151 = Greater?(x=w651, y=w652) -> (0:→"Behav Cam":bool)
        n152 = Subtract(x=w656, y=w650) -> (x-y=w657:u32)
        n153 = Divide(x=w657, y=u32 1000) -> (x/y=w646:dbl)
        n154 = call "GrabWebCam_2P.vi"("Session In"=w644, "Image In"=w645, "Trial Time"=w646, "AVI Refnum"=w647, "error in"=w648) -> ("Session Out"=w638:T3, "WebCam Img Out"=→"?":T1, "Buffer Number Out"=w642:u32, "error out"=w649:errorcluster)  [unwired: 7 in]
        n155 = call <vilib>:"Calculate Frames per Second.vi"("Update Interval (ms)"=u32 5000, "Buffer Number"=w642) -> ("Processed Frames/s"=→"Behavior Cam Fs":dbl)  [unwired: 7 in, 2 out]
        n156 = local read "Analog Data"() -> (w641:bool)
        n157 = local read "stop"() -> (w639:bool)
        n158 = Compound Arithmetic op=OR(w639, w641) -> (w640:bool)
      }
      n159 = while {
        tunnel: [w623] -> w359
        tunnel: [w630] -> w361
        tunnel: w408 -> [w622]
        tunnel: w407 -> [w621]
        tunnel: w406 -> [w620]
        tunnel: w405 -> [w619]
        tunnel: w402 -> [w618]
        tunnel: [w617] -> w360
        tunnel: w400 -> [w617]
        i -> [w631]
        stop <- w625 stop-if-true
        n160 = Tick Count (ms)() -> (millisecond timer value=w635:u32)
        n161 = Greater?(x=w621, y=w631) -> (0:→"MScan Cam":bool)
        n162 = Subtract(x=w635, y=w622) -> (x-y=w636:u32)
        n163 = Divide(x=w636, y=u32 1000) -> (x/y=w629:dbl)
        n164 = call "GrabWebCam_2P.vi"("Session In"=w620, "Image In"=w618, "Trial Time"=w629, "AVI Refnum"=w617, "error in"=w619) -> ("Session Out"=w623:T3, "WebCam Img Out"=→"?":T1, "Buffer Number Out"=w627:u32, "error out"=w630:errorcluster)  [unwired: 7 in]
        n165 = call <vilib>:"Calculate Frames per Second.vi"("Update Interval (ms)"=u32 5000, "Buffer Number"=w627) -> ("Processed Frames/s"=→"MSCan Cam Fs":dbl)  [unwired: 7 in, 2 out]
        n166 = local read "Analog Data"() -> (w626:bool)
        n167 = local read "stop"() -> (w624:bool)
        n168 = Compound Arithmetic op=OR(w624, w626) -> (w625:bool)
      }
      n169 = flat-sequence {
        tunnel: [w597] -> w385
        tunnel: [w596] -> w384
        tunnel: w383 -> [w586]
        tunnel: w382 -> [w595]
        tunnel: w381 -> [w594]
        tunnel: w380 -> [w593]
        tunnel: [w592] -> w379
        tunnel: [w591] -> w378
        tunnel: [w590] -> w377
        tunnel: [w589] -> w376
        tunnel: w375 -> [w588]
        tunnel: w331 -> [w587]
        tunnel: w366 -> [w585]
        tunnel: w365 -> [w584]
        tunnel: w364 -> [w582]
        tunnel: w363 -> [w583]
        tunnel: w362 -> [w581]
        tunnel: w361 -> [w579]
        tunnel: w360 -> [w580]
        tunnel: w359 -> [w578]
        tunnel: [w577] -> w358
        tunnel: [w576] -> w356
        tunnel: [w575] -> w347
        tunnel: w346 -> [w575]
        tunnel: [w574] -> w344
        tunnel: w343 -> [w574]
        tunnel: [w573] -> w341
        tunnel: w340 -> [w573]
        tunnel: [w572] -> w338
        tunnel: w337 -> [w572]
        tunnel: [w571] -> w335
        tunnel: w334 -> [w571]
        tunnel: [w570] -> w332
        tunnel: w331 -> [w570]
        tunnel: w327 -> [w569]
        tunnel: [w569] -> w329
        tunnel: w326 -> [w568]
        tunnel: [w568] -> w328
        tunnel: w385 -> [w613]
        tunnel: w384 -> [w612]
        tunnel: w379 -> [w611]
        tunnel: w378 -> [w610]
        tunnel: w377 -> [w609]
        tunnel: w376 -> [w608]
        tunnel: w358 -> [w607]
        tunnel: [w607] -> w357
        tunnel: w356 -> [w606]
        tunnel: [w606] -> w355
        tunnel: w347 -> [w605]
        tunnel: [w605] -> w345
        tunnel: w344 -> [w604]
        tunnel: [w604] -> w342
        tunnel: w341 -> [w603]
        tunnel: [w603] -> w339
        tunnel: w338 -> [w602]
        tunnel: [w602] -> w336
        tunnel: w335 -> [w601]
        tunnel: [w601] -> w333
        tunnel: w332 -> [w600]
        tunnel: [w600] -> w330
        tunnel: w329 -> [w599]
        tunnel: [w599] -> w324
        tunnel: [w598] -> w325
        tunnel: w328 -> [w598]
        frame #0 {
          n170 = call <vilib>:"DAQmx Stop Task.vi"("task/channels in"=w586, "error in"=w595) -> ("task out"=w597:refnum<k21>, "error out"=w596:errorcluster)  [unwired: 12 in]
          n171 = call <vilib>:"DAQmx Stop Task.vi"("task/channels in"=w594, "error in"=w593) -> ("task out"=w591:refnum<k21>, "error out"=w592:errorcluster)  [unwired: 12 in]
          n172 = call <vilib>:"IMAQdx Close Camera.vi"("error in"=w585, "Session In"=w584) -> ()  [unwired: 9 in, 1 out]
          n173 = call <vilib>:"IMAQdx Close Camera.vi"("error in"=w582, "Session In"=w581) -> ()  [unwired: 9 in, 1 out]
          n174 = call "IMAQ AVI2 Close"("error in (no error)"=w582, "AVI Refnum"=w583) -> ("error out"=w577:errorcluster)  [unwired: 9 in]
          n175 = call <vilib>:"IMAQdx Close Camera.vi"("error in"=w579, "Session In"=w578) -> ()  [unwired: 9 in, 1 out]
          n176 = call "IMAQ AVI2 Close"("error in (no error)"=w579, "AVI Refnum"=w580) -> ("error out"=w576:errorcluster)  [unwired: 9 in]
          n177 = call <vilib>:"DAQmx Stop Task.vi"("task/channels in"=w588, "error in"=w587) -> ("task out"=w590:refnum<k21>, "error out"=w589:errorcluster)  [unwired: 12 in]
        }
        frame #1 {
          n178 = call <vilib>:"DAQmx Clear Task.vi"("task in"=w613, "error in"=w612) -> ()  [unwired: 13 in, 1 out]
          n179 = call <vilib>:"DAQmx Clear Task.vi"("task in"=w610, "error in"=w611) -> ()  [unwired: 13 in, 1 out]
          n180 = call <vilib>:"DAQmx Clear Task.vi"("task in"=w609, "error in"=w608) -> ()  [unwired: 13 in, 1 out]
        }
      }
      n181 = Delete From Array(array=w342, length=1, index=0) -> (array with subset deleted=w552:u32[])  [unwired: 1 out]
      n182 = Delete From Array(array=w345, length=1, index=0) -> (array with subset deleted=w553:u32[])  [unwired: 1 out]
      n183 = Close File(refnum=w336, error in=w339) -> (path=w527:path, error out=w528:errorcluster)
      n184 = Move(source path=w324, error in=w357, 10:"Target Path") -> (error out=w449:errorcluster)  [unwired: 2 in, 2 out]
      n185 = Move(source path=w325, error in=w355, 10:"Target Path") -> (error out=w401:errorcluster)  [unwired: 2 in, 2 out]
      n186 = Move(source path=w527, error in=w528, 10:"Target Path") -> (error out=w530:errorcluster)  [unwired: 2 in, 2 out]
      n187 = Build Array(w553, w552) -> (w550:u32[][])
      n188 = call <vilib>:"Simple Error Handler.vi"("error in (no error)"=w449) -> ()  [unwired: 1 in, 8 out]
      n189 = call <vilib>:"Simple Error Handler.vi"("error in (no error)"=w401) -> ()  [unwired: 1 in, 8 out]
      n190 = Array To Spreadsheet String(delimiter (Tab)=",", array=w553, 3:"%d" ("format string")) -> (spreadsheet string=w543:string)
      n191 = Array To Spreadsheet String(delimiter (Tab)=",", array=w552, 3:"%d" ("format string")) -> (spreadsheet string=w544:string)
      n192 = Transpose 2D Array(2D array=w550) -> (transposed array=w551:u32[][])
      n193 = call <vilib>:"Simple Error Handler.vi"("error in (no error)"=w530) -> ()  [unwired: 1 in, 8 out]
      n194 = call <vilib>:"Trim Whitespace.vi"("string"=w543) -> ("trimmed string"=w425:string)  [unwired: 1 in]
      n195 = call <vilib>:"Trim Whitespace.vi"("string"=w544) -> ("trimmed string"=w545:string)  [unwired: 1 in]
      n196 = Number To Decimal String(number=w551) -> ()  [unwired: 1 in, 1 out]
      n197 = Build Array(w425, w545) -> (w546:string[])
      n198 = TDMS Set Properties(5:w546, 7:string[] ["WhiskerCam_DroppedFrameIndex", "WhiskerCam_NumberDropped"] ("channel name(s) in (Untitled)"), 8:w330, 11:w333) -> (0:w541:errorcluster, 3:w542:refnum<k34>)  [unwired: 2 in, 2 out]
      n199 = TDMS Close(8:w541, 11:w542) -> (0:w526:errorcluster, 3:w531:path)
      n200 = Path To String(path=w531) -> (string=w424:string)
      n201 = TDMS Defragment(4:w526, 7:w531) -> (0:w534:errorcluster)
      n202 = Concatenate Strings(w424, "_index" ("string")) -> (w532:string)
      n203 = String To Path(string=w532) -> (path=w533:path)
      n204 = Move(source path=w531, error in=w534, 10:"Target Path") -> (error out=w529:errorcluster)  [unwired: 2 in, 2 out]
      n205 = Move(source path=w533, error in=w534, 10:"Target Path") -> (error out=w423:errorcluster)  [unwired: 2 in, 2 out]
      n206 = call <vilib>:"Simple Error Handler.vi"("error in (no error)"=w423) -> ()  [unwired: 1 in, 8 out]
      n207 = call <vilib>:"Simple Error Handler.vi"("error in (no error)"=w529) -> ()  [unwired: 1 in, 8 out]
    }
    frame #4 {
      "Complete" <- TRUE ("Data Acquisition - Complete")
    }
  }
